vi "UHR-Fleezers Control (host) - 12.7e.vi"() -> ()   [LabVIEW 2012] (continued)
                      n1710 = Greater?(x=w2546, y="Stop F (pN) (mask)") -> (0:w2544:bool[])
                      n1711 = Or Array Elements(Boolean array=w2557) -> (logical OR=w2542:bool)
                      n1712 = Or Array Elements(Boolean array=w2544) -> (logical OR=w2541:bool)
                      n1713 = Greater?(x=w2551, y="Attempt Limit") -> (0:w2553:bool)
                      n1714 = case shown="True" w2553 {
                        frame False {
                        }
                        frame True {
                          n1715 = local write "Fish for Tether"(FALSE ("Fish for Tether")) -> ()
                          n1716 = call <vilib>:"Beep.vi"() -> ()  [unwired: 3 in, 9 out]
                          n1717 = local read "Messages"() -> (w2569:string)
                          n1718 = call "Update messages.vi"("Message to add"="Tether fishing timeout." ("Messages"), "Old message string"=w2569) -> ("New message string"=→"Messages":string)
                        }
                      }
                      n1719 = Select(t=w2542, s="Normal (on) or masked test (off)", f=w2541) -> (s? t:f=w2540:bool)
                    }
                  }
                  n1720 = local read "BD 2 Frequency 1 (MHz)"() -> (w2516:dbl)
                  n1721 = Select(t=w2517, s="Scan axis 2", f=w2516) -> (s? t:f=w2520:dbl)
                  n1722 = Add(x=w2508, y=w2520) -> (x+y=w2514:dbl)
                  n1723 = Select(t=w2514, s="Scan axis 2", f=w2517) -> (s? t:f=w2523:dbl)
                  n1724 = Select(t=w2516, s="Scan axis 2", f=w2514) -> (s? t:f=w2522:dbl)
                  n1725 = local read "BD 2 Frequency 2 (MHz)"() -> (w2525:dbl)
                  n1726 = local read "BD 2 Frequency 3 (MHz)"() -> (w2524:dbl)
                  n1727 = local read "Y RF Frequency Limits (MHz)"() -> (w2518:T16)
                  n1728 = local read "X RF Frequency Limits (MHz)"() -> (w2519:T16)
                  n1729 = local read "BD 1 Frequency 3 (MHz)"() -> (w2526:dbl)
                  n1730 = call "set RF board frequency - interlace.vi"("Board 2 Frequency Limits"=w2518, "Board 1 Frequency Limits"=w2519, "FPGA VI Reference In"=w2506, "Board 2 Frequency 3 (MHz)"=w2524, "Board 1 Frequency 3 (MHz)"=w2526, "Board 2 Frequency 2 (MHz)"=w2525, "Board 2 Frequency 1 (MHz)"=w2522, "Board 1 Frequency 2 (MHz)"=w2509, "Board 1 Frequency 1  (MHz)"=w2523) -> ()  [unwired: 1 in, 2 out]
                }
                frame #1 {
                  n1731 = And(x=w2577, y=w2574) -> (x .and. y?=w2576:bool)
                  n1732 = case "Only if were fishing and now formed tether" shown="True" w2576 {
                    tunnel: w2575 -> [w2579 w2594]
                    tunnel: [w2578 w2593] -> w2573
                    tunnel: w2572 -> [_ w2589]
                    frame False {
                      n1733 = local read "Fish for Tether"() -> (w2578:bool)
                      n1734 = case shown="False" w2578 {
                        tunnel: w2579 -> [w2580 _]
                        frame False {
                          n1735 = property on="BD 1 Frequency 1 (MHz)" class="DigNum (strict)"("Val(Sgnl)"=w2580) -> ()  [unwired: 2 in, 2 out]
                        }
                        frame True {
                        }
                      }
                    }
                    frame True {
                      w2593 = FALSE ("Fish for Tether")
                      n1736 = call <vilib>:"Beep.vi"() -> ()  [unwired: 3 in, 9 out]
                      n1737 = Number To Decimal String(number=w2589, width (-)=i16 1) -> (decimal integer string=w2587:string)
                      n1738 = Concatenate Strings("Formed tether in ", w2587, " attempt(s)." ("string")) -> (w2584:string)
                      n1739 = local read "Messages"() -> (w2591:string)
                      n1740 = local write "Fish for Tether"(w2593) -> ()
                      n1741 = call "Update messages.vi"("Message to add"=w2584, "Old message string"=w2591) -> ("New message string"=w2590:string)
                      n1742 = local write "Messages"(w2590) -> ()
                      n1743 = Get Date/Time In Seconds() -> (seconds since 1Jan1904=→"Time tether formed":timestamp)
                      n1744 = local read "Flow ON during cal?"() -> (w2581:bool)
                      n1745 = property on="Sample Channel\nFlow" class="Bool (strict)"("Val(Sgnl)"=w2581) -> (error out=w2582:errorcluster)  [unwired: 2 in, 1 out]
                      n1746 = case shown="\"2\", \"3\", \"4\", \"5\", \"6\"" "Then..." {
                        selector: "Then..." -> [_ w2597]
                        tunnel: w2594 -> [w2596 _]
                        tunnel: w2582 -> [_ _]
                        frame "1", Default {
                          n1747 = property on="BD 1 Frequency 1 (MHz)" class="DigNum (strict)"("Val(Sgnl)"=w2596) -> ()  [unwired: 2 in, 2 out]
                        }
                        frame "2", "3", "4", "5", "6" {
                          n1748 = flat-sequence {
                            tunnel: w2597 -> [w2599]
                            frame #0 {
                              n1749 = property on="Trap Delta (MHz)" class="DigNum (strict)"("Val(Sgnl)"="Move to Delta 1 (MHz)") -> ()  [unwired: 2 in, 2 out]
                            }
                            frame #1 {
                              n1750 = case shown="\"5\", \"6\"" w2599 {
                                selector: w2599 -> [w2602 w2612 _]
                                frame "3", "4" {
                                n1751 = flat-sequence {
                                tunnel: w2602 -> [w2603]
                                tunnel: [w2603] -> w2600
                                tunnel: [w2605] -> w2601
                                tunnel: w2600 -> [w2605]
                                tunnel: w2601 -> [w2609]
                                frame #0 {
                                n1752 = property on="Green Laser ON" class="Bool (strict)"("Val(Sgnl)"=TRUE ("Value (Signaling)")) -> ()  [unwired: 2 in, 2 out]
                                }
                                frame #1 {
                                n1753 = Multiply(x="Wait Before Save (s)", y=u32 1000 ("x")) -> (x*y=w2607:u32)
                                n1754 = Wait (ms)(milliseconds to wait=w2607) -> ()  [unwired: 1 out]
                                }
                                frame #2 {
                                n1755 = property on="Start Saving" class="Bool (strict)"("Value"=TRUE ("Start Saving")) -> ()  [unwired: 2 in, 2 out]
                                n1756 = case shown="\"4\"" w2609 {
                                frame Default {
                                }
                                frame "4" {
                                n1757 = property on="Fl. Triggered..." class="Bool (strict)"("Val(Sgnl)"=TRUE ("Value (Signaling)")) -> ()  [unwired: 2 in, 2 out]
                                }
                                }
                                }
                                }
                                }
                                frame "5", "6" {
                                n1758 = stacked-sequence {
                                tunnel: w2612 -> [_ _ _ _ _ _ w2624]
                                frame #0 {
                                n1759 = Replace Array Subset(array=u32[] [0] ("Index Values"), new element="Raster Set Upon Tether", index=0) -> (w2613:u32[])
                                n1760 = property on="Saved AOD Raster Scan Parameter Sets" class="Arr (strict)"("Index Values"=w2613) -> ()  [unwired: 2 in, 2 out]
                                }
                                frame #1 {
                                n1761 = Wait (ms)(milliseconds to wait=u32 500) -> ()  [unwired: 1 out]
                                }
                                frame #2 {
                                n1762 = property on="Load parameters" class="Bool (strict)"("Val(Sgnl)"=TRUE ("Value (Signaling)")) -> ()  [unwired: 2 in, 2 out]
                                n1763 = case shown="True" "Green ON During Raster" {
                                frame False {
                                }
                                frame True {
                                n1764 = property on="Green Laser ON" class="Bool (strict)"("Val(Sgnl)"=TRUE ("Value (Signaling)")) -> ()  [unwired: 2 in, 2 out]
                                }
                                }
                                }
                                frame #3 {
                                n1765 = Wait (ms)(milliseconds to wait=u32 500) -> ()  [unwired: 1 out]
                                }
                                frame #4 {
                                n1766 = property on="Trap Raster Scan" class="Bool (strict)"("Val(Sgnl)"=TRUE ("Value (Signaling)")) -> ()  [unwired: 2 in, 2 out]
                                }
                                frame #5 {
                                n1767 = Wait (ms)(milliseconds to wait=u32 2000) -> ()  [unwired: 1 out]
                                }
                                frame #6 {
                                n1768 = flat-sequence {
                                tunnel: w2624 -> [w2631]
                                frame #0 {
                                n1769 = while {
                                stop <- w2627 stop-if-true
                                n1770 = local read "Raster Scanning..."() -> (w2626:bool)
                                n1771 = local read "Saving..."() -> (w2629:bool)
                                n1772 = Wait (ms)(milliseconds to wait=u32 100) -> ()  [unwired: 1 out]
                                n1773 = Not(x=w2629) -> (.not. x?=w2628:bool)
                                n1774 = Not(x=w2626) -> (.not. x?=w2625:bool)
                                n1775 = And(x=w2628, y=w2625) -> (x .and. y?=w2627:bool)
                                }
                                }
                                frame #1 {
                                n1776 = local read "Tether"() -> (w2632:bool)
                                n1777 = case shown="True" w2632 {
                                tunnel: w2631 -> [_ w2634]
                                frame False {
                                n1778 = property on="Fish for Tether" class="Bool (strict)"("Val(Sgnl)"="Fish again after \nraster break?") -> ()  [unwired: 2 in, 2 out]
                                }
                                frame True {
                                n1779 = stacked-sequence {
                                tunnel: w2634 -> [_ w2638 _ _]
                                frame #0 {
                                n1780 = property on="Trap Delta (MHz)" class="DigNum (strict)"("Val(Sgnl)"="Move to Delta 2 (MHz)") -> ()  [unwired: 2 in, 2 out]
                                n1781 = case shown="True" "Flow ON after\ntether testing?" {
                                frame False {
                                }
                                frame True {
                                n1782 = property on="Sample Channel\nFlow" class="Bool (strict)"("Val(Sgnl)"=TRUE ("Value (Signaling)")) -> ()  [unwired: 2 in, 2 out]
                                }
                                }
                                }
                                frame #1 {
                                n1783 = flat-sequence {
                                tunnel: w2638 -> [w2640]
                                frame #0 {
                                n1784 = Wait (ms)(milliseconds to wait=u32 500) -> ()  [unwired: 1 out]
                                }
                                frame #1 {
                                n1785 = case shown="\"6\"" w2640 {
                                frame Default {
                                }
                                frame "6" {
                                n1786 = property on="Green Laser ON" class="Bool (strict)"("Val(Sgnl)"=TRUE ("Green Laser ON/Interlacing")) -> ()  [unwired: 2 in, 2 out]
                                }
                                }
                                }
                                frame #2 {
                                n1787 = Wait (ms)(milliseconds to wait=u32 500) -> ()  [unwired: 1 out]
                                }
                                frame #3 {
                                n1788 = local write "Start Saving"("Save at end (5, 6)") -> ()
                                }
                                }
                                }
                                frame #2 {
                                n1789 = local read "Bead Sep. Int. Time (s)"() -> (w2646:dbl)
                                n1790 = Multiply(x=w2646, y=1000.0) -> (x*y=w2645:dbl)
                                n1791 = Wait (ms)(milliseconds to wait=w2645) -> ()  [unwired: 1 out]
                                }
                                frame #3 {
                                n1792 = property on="Remove Offset" class="Bool (strict)"("Val(Sgnl)"=TRUE ("Value (Signaling)")) -> ()  [unwired: 2 in, 2 out]
                                }
                                }
                                }
                                }
                                }
                                }
                                }
                                }
                                }
                                frame "2", Default {
                                }
                              }
                            }
                          }
                        }
                      }
                      "Tether" <- "Tether Alarm?"
                    }
                  }
                }
                frame #2 {
                  n1793 = local read "Oscillate Set 1"() -> (w2653:bool)
                  n1794 = local read "Stop All"() -> (w2651:bool)
                  n1795 = Or(x=w2653, y=w2648) -> (x .or. y?=w2650:bool)
                  n1796 = Not(x=w2650) -> (.not. x?=w2652:bool)
                  n1797 = Compound Arithmetic op=OR(w2651, w2652) -> (w2649:bool)
                }
              }
              n1798 = node-c288() -> ()  [unwired: 2 out]
            }
            n1799 = node-c288(w2485) -> ()  [unwired: 1 out]
          }
        }
      }
      event "Fl. Triggered...": Value Change {
        n1800 = event-data() -> ()  [unwired: 7 out]
        n1801 = case shown="True" "Fl. Triggered..." {
          frame False {
          }
          frame True {
            n1802 = node-c288() -> (w2664:T23)  [unwired: 4 out]
            n1803 = timed-loop {
              timing: w2664 -> [_]
              timing-out: [_] -> w2663
              tunnel: "Action" -> [w2672]
              shift-right: [w2669] -> _
              shift-left: u8 255 -> [w2671]
              shift-right: [w2666] -> _
              shift-left: 255 -> [w2668]
              stop <- w2665 stop-if-true
              # "Reset confocal spot"
              n1804 = node-c288() -> ()  [unwired: 2 out]
              n1805 = flat-sequence {
                tunnel: w2672 -> [w2692]
                tunnel: w2671 -> [w2691]
                tunnel: [w2690] -> w2670
                tunnel: w2668 -> [w2677]
                tunnel: [w2676] -> w2667
                tunnel: [w3071] -> w2665
                tunnel: w2670 -> [w3070]
                tunnel: [w3070] -> w2669
                tunnel: [w3069] -> w2666
                tunnel: w2667 -> [w3069]
                frame #0 {
                  n1806 = local read "Delta Fl. 2"() -> (w2689:dbl)
                  n1807 = local read "Delta Fl. 1"() -> (w2684:dbl)
                  n1808 = Multiply(x="Fl. Delta Thresh. (kHz)", y=1000.0) -> (x*y=w2679:dbl)
                  n1809 = Select(t=w2684, s="APD to Watch", f=w2689) -> (s? t:f=w2680:dbl)
                  n1810 = Greater?(x=w2680, y=w2679) -> (0:w2685:bool)
                  n1811 = Or(x="Force Yank", y=w2685) -> (x .or. y?=w2683:bool)
                  n1812 = And(x=w2683, y="Yank when?") -> (x .and. y?=w2681:bool)
                  n1813 = case shown="False" w2681 {
                    tunnel: w2692 -> [w2695 w2896]
                    tunnel: w2691 -> [w2697 w2892]
                    tunnel: [w2697 w2890] -> w2690
                    tunnel: w2680 -> [w2703 _]
                    tunnel: w2679 -> [w2702 _]
                    tunnel: "Force Yank" -> [w2700 _]
                    tunnel: w2677 -> [w2699 w2889]
                    tunnel: [w2698 w2889] -> w2676
                    frame False {
                      n1814 = Negate(x=w2702) -> (-x=w2694:dbl)
                      n1815 = local write "Fl. High"(TRUE ("Fl. High")) -> ()
                      n1816 = Less?(x=w2703, y=w2694) -> (x < y?=w2701:bool)
                      n1817 = Or(x=w2700, y=w2701) -> (x .or. y?=w2696:bool)
                      n1818 = case shown="True" w2696 {
                        tunnel: w2699 -> [w2704 w2714]
                        tunnel: [w2704 w2713] -> w2698
                        tunnel: w2695 -> [_ w2712]
                        frame False {
                        }
                        frame True {
                          n1819 = flat-sequence {
                            tunnel: w2714 -> [w2720]
                            tunnel: w2712 -> [w2717]
                            tunnel: [w2719] -> w2711
                            tunnel: [w2718] -> w2710
                            tunnel: [w2717] -> w2709
                            tunnel: w2708 -> [w2716]
                            tunnel: [w2716] -> w2707
                            tunnel: w2706 -> [w2715]
                            tunnel: [w2715] -> w2705
                            tunnel: [w2791] -> w2713
                            tunnel: w2711 -> [w2791]
                            tunnel: w2710 -> [w2790]
                            tunnel: w2709 -> [w2789]
                            tunnel: w2707 -> [w2788]
                            tunnel: w2705 -> [w2787]
                            frame #0 {
                              n1820 = call <vilib>:"Beep.vi"() -> ()  [unwired: 12 in]
                              n1821 = local write "Waiting"(FALSE ("Waiting")) -> ()
                              n1822 = Increment(x=w2720) -> (x+1=w2719:i32)
                              n1823 = case shown="\"Image\"" w2717 {
                                tunnel: w2719 -> [_ w2725 _]
                                frame "Alarm", Default {
                                }
                                frame "Yank" {
                                n1824 = flat-sequence {
                                tunnel: w2725 -> [w2728]
                                tunnel: [w2727] -> w2724
                                tunnel: [w2726] -> w2723
                                tunnel: w2724 -> [w2738]
                                tunnel: w2723 -> [w2739]
                                frame #0 {
                                n1825 = local read "Yank Delay (s)"() -> (w2731:dbl)
                                n1826 = local read "N Array El"() -> (w2726:u8)
                                n1827 = Quotient & Remainder(x=w2728, y=w2726) -> (x-y*floor(x/y)=w2727:i32)  [unwired: 1 out]
                                n1828 = Multiply(x=w2731, y=1000.0) -> (x*y=w2729:dbl)
                                n1829 = Wait (ms)(milliseconds to wait=w2729) -> ()  [unwired: 1 out]
                                }
                                frame #1 {
                                n1830 = local read "Yank to which?"() -> (w2733:bool)
                                n1831 = local read "Random Choice"() -> (w2743:bool)
                                n1832 = local read "Yank to Trap Delta (MHz)"() -> (w2736:dbl[])
                                n1833 = local read "Yank to SP"() -> (w2737:dbl[])
                                n1834 = Random Number (0-1)() -> (number: 0 to 1=w2742:dbl)
                                n1835 = Multiply(x=w2739, y=w2742) -> (x*y=w2741:dbl)
                                n1836 = Round Toward -Infinity(1:w2741) -> (0:w2740:dbl)
                                n1837 = Select(t=w2740, s=w2743, f=w2738) -> (s? t:f=w2734:dbl)
                                n1838 = Select(t=w2736, s=w2733, f=w2737) -> (s? t:f=w2735:dbl[])
                                n1839 = Index Array(array=w2735, index=w2734) -> (element=w2732:dbl)
                                n1840 = case shown="True" w2733 {
                                tunnel: w2732 -> [w2744 w2771]
                                frame False {
                                n1841 = flat-sequence {
                                tunnel: w2744 -> [w2745]
                                frame #0 {
                                n1842 = property on="Trap Pos FB SP" class="DigNum (strict)"("Val(Sgnl)"=w2745) -> ()  [unwired: 2 in, 2 out]
                                }
                                frame #1 {
                                n1843 = Wait (ms)(milliseconds to wait=u32 700) -> ()  [unwired: 1 out]
                                }
                                frame #2 {
                                n1844 = local read "Action (%)"() -> (w2750:dbl)
                                n1845 = Absolute Value(x=w2750) -> (abs(x)=w2749:dbl)
                                n1846 = Greater?(x=w2749, y=70.0) -> (0:w2747:bool)
                                n1847 = property on="Remove Action Offset" class="Bool (strict)"("Val(Sgnl)"=w2747) -> ()  [unwired: 2 in, 2 out]
                                }
                                frame #3 {
                                n1848 = for {
                                N: 4 -> [_]
                                n1849 = flat-sequence {
                                frame #0 {
                                n1850 = Wait (ms)(milliseconds to wait=u32 500) -> ()  [unwired: 1 out]
                                }
                                frame #1 {
                                n1851 = local read "Action (%)"() -> (w2756:dbl)
                                n1852 = Absolute Value(x=w2756) -> (abs(x)=w2755:dbl)
                                n1853 = Greater?(x=w2755, y=70.0) -> (0:w2753:bool)
                                n1854 = property on="Remove Action Offset" class="Bool (strict)"("Val(Sgnl)"=w2753) -> ()  [unwired: 2 in, 2 out]
                                }
                                }
                                }
                                }
                                frame #4 {
                                n1855 = Wait (ms)(milliseconds to wait=u32 500) -> ()  [unwired: 1 out]
                                }
                                frame #5 {
                                n1856 = local read "Mean"() -> (w2764:dbl)
                                n1857 = Greater?(x=w2764, y=11.0) -> (0:w2758:bool)
                                n1858 = Not(x=w2758) -> (.not. x?=w2759:bool)
                                n1859 = And(x=w2759, y="Shift confocal") -> (x .and. y?=w2761:bool)
                                n1860 = And(x=w2758, y="Shift confocal") -> (x .and. y?=w2762:bool)
                                n1861 = case shown="True" w2762 {
                                frame False {
                                }
                                frame True {
                                n1862 = local read "Confocal Y 2 (V)"() -> (w2768:dbl)
                                n1863 = local read "Confocal X 2 (V)"() -> (w2767:dbl)
                                n1864 = property on="AO1" class="Slide (strict)"("Val(Sgnl)"=w2768) -> ()  [unwired: 2 in, 2 out]
                                n1865 = property on="AO2" class="Slide (strict)"("Val(Sgnl)"=w2767) -> ()  [unwired: 2 in, 2 out]
                                }
                                }
                                n1866 = case shown="True" w2761 {
                                frame False {
                                }
                                frame True {
                                n1867 = local read "Confocal Y 1 (V)"() -> (w2766:dbl)
                                n1868 = local read "Confocal X 1 (V)"() -> (w2765:dbl)
                                n1869 = property on="AO1" class="Slide (strict)"("Val(Sgnl)"=w2766) -> ()  [unwired: 2 in, 2 out]
                                n1870 = property on="AO2" class="Slide (strict)"("Val(Sgnl)"=w2765) -> ()  [unwired: 2 in, 2 out]
                                }
                                }
                                }
                                frame #6 {
                                n1871 = Wait (ms)(milliseconds to wait=u32 1500) -> ()  [unwired: 1 out]
                                }
                                frame #7 {
                                n1872 = property on="Rem fb disp offset" class="Bool (strict)"("Val(Sgnl)"=TRUE ("Value (Signaling)")) -> ()  [unwired: 2 in, 2 out]
                                }
                                }
                                }
                                frame True {
                                n1873 = flat-sequence {
                                tunnel: w2771 -> [w2772]
                                frame #0 {
                                n1874 = property on="Trap Delta (MHz)" class="DigNum (strict)"("Val(Sgnl)"=w2772) -> ()  [unwired: 2 in, 2 out]
                                }
                                frame #1 {
                                n1875 = Wait (ms)(milliseconds to wait=u32 500) -> ()  [unwired: 1 out]
                                }
                                frame #2 {
                                n1876 = local read "Shift confocal"() -> (w2778:bool)
                                n1877 = local read "Mean"() -> (w2780:dbl)
                                n1878 = Greater?(x=w2780, y=11.0) -> (0:w2777:bool)
                                n1879 = Not(x=w2777) -> (.not. x?=w2776:bool)
                                n1880 = And(x=w2776, y=w2778) -> (x .and. y?=w2774:bool)
                                n1881 = And(x=w2777, y=w2778) -> (x .and. y?=w2775:bool)
                                n1882 = case shown="True" w2775 {
                                frame False {
                                }
                                frame True {
                                n1883 = local read "Confocal Y 2 (V)"() -> (w2784:dbl)
                                n1884 = local read "Confocal X 2 (V)"() -> (w2783:dbl)
                                n1885 = property on="AO2" class="Slide (strict)"("Val(Sgnl)"=w2783) -> ()  [unwired: 2 in, 2 out]
                                n1886 = property on="AO1" class="Slide (strict)"("Val(Sgnl)"=w2784) -> ()  [unwired: 2 in, 2 out]
                                }
                                }
                                n1887 = case shown="True" w2774 {
                                frame False {
                                }
                                frame True {
                                n1888 = local read "Confocal X 1 (V)"() -> (w2781:dbl)
                                n1889 = local read "Confocal Y 1 (V)"() -> (w2782:dbl)
                                n1890 = property on="AO2" class="Slide (strict)"("Val(Sgnl)"=w2781) -> ()  [unwired: 2 in, 2 out]
                                n1891 = property on="AO1" class="Slide (strict)"("Val(Sgnl)"=w2782) -> ()  [unwired: 2 in, 2 out]
                                }
                                }
                                }
                                }
                                }
                                }
                                }
                                }
                                }
                                frame "Image" {
                                n1892 = property on="Confocal Image" class="Bool (strict)"("Val(Sgnl)"=TRUE ("Value (Signaling)")) -> ()  [unwired: 2 in, 2 out]
                                }
                              }
                              n1893 = local write "Fl. High"(FALSE ("Fl. High")) -> ()
                              n1894 = local read "Time (s)"() -> (w2718:dbl)
                            }
                            frame #1 {
                              n1895 = case shown="True" "Auto F Reset" {
                                tunnel: w2790 -> [_ w2795]
                                tunnel: w2789 -> [_ w2794]
                                tunnel: w2788 -> [_ w2793]
                                tunnel: w2787 -> [_ w2792]
                                frame False {
                                }
                                frame True {
                                n1896 = node-c288() -> (w2797:T23)  [unwired: 4 in]
                                n1897 = timed-loop {
                                timing: w2797 -> [_]
                                timing-out: [_] -> w2796
                                tunnel: w2795 -> [w2802]
                                tunnel: w2794 -> [w2801]
                                tunnel: w2793 -> [w2800]
                                tunnel: w2792 -> [w2799]
                                stop <- w2798 stop-if-true
                                n1898 = node-c288() -> ()  [unwired: 1 in, 1 out]
                                n1899 = local read "Fl. Delta Thresh. (kHz)"() -> (w2811:dbl)
                                n1900 = local read "APD to Watch"() -> (w2812:bool)
                                n1901 = local read "Delta Fl. 1"() -> (w2813:dbl)
                                n1902 = local read "Delta Fl. 2"() -> (w2814:dbl)
                                n1903 = local read "Fl. Triggered..."() -> (w2805:bool)
                                n1904 = local read "Stop All"() -> (w2806:bool)
                                n1905 = local read "Reset Force"() -> (w2804:bool)
                                n1906 = Multiply(x=w2811, y=1000.0) -> (x*y=w2809:dbl)
                                n1907 = Select(t=w2813, s=w2812, f=w2814) -> (s? t:f=w2808:dbl)
                                n1908 = Not(x=w2805) -> (.not. x?=w2803:bool)
                                n1909 = Greater?(x=w2808, y=w2809) -> (0:w2807:bool)
                                n1910 = Compound Arithmetic op=OR(w2807, w2806, w2803, w2804) -> (w2798:bool)
                                n1911 = case shown="True" w2798 {
                                tunnel: w2802 -> [_ w2818]
                                tunnel: w2801 -> [_ w2822]
                                tunnel: w2800 -> [_ w2821]
                                tunnel: w2799 -> [_ w2820]
                                frame False {
                                }
                                frame True {
                                n1912 = case shown="\"Yank\"" w2822 {
                                tunnel: w2821 -> [_ w2832]
                                tunnel: w2820 -> [_ w2830]
                                frame "Image", Default {
                                }
                                frame "Yank" {
                                n1913 = flat-sequence {
                                tunnel: [w2835] -> w2833
                                tunnel: w2832 -> [w2835]
                                tunnel: [w2834] -> w2831
                                tunnel: w2830 -> [w2834]
                                tunnel: w2833 -> [w2841]
                                tunnel: w2831 -> [w2839]
                                frame #0 {
                                n1914 = local read "Yank Delay (s)"() -> (w2838:dbl)
                                n1915 = Multiply(x=w2838, y=1000.0) -> (x*y=w2836:dbl)
                                n1916 = Wait (ms)(milliseconds to wait=w2836) -> ()  [unwired: 1 out]
                                }
                                frame #1 {
                                n1917 = local read "Yank to which?"() -> (w2840:bool)
                                n1918 = case shown="False" w2840 {
                                tunnel: w2841 -> [_ w2869]
                                tunnel: w2839 -> [w2842 _]
                                frame False {
                                n1919 = flat-sequence {
                                tunnel: w2842 -> [w2843]
                                frame #0 {
                                n1920 = property on="Trap Pos FB SP" class="DigNum (strict)"("Val(Sgnl)"=w2843) -> ()  [unwired: 2 in, 2 out]
                                }
                                frame #1 {
                                n1921 = Wait (ms)(milliseconds to wait=u32 700) -> ()  [unwired: 1 out]
                                }
                                frame #2 {
                                n1922 = local read "Action (%)"() -> (w2848:dbl)
                                n1923 = Absolute Value(x=w2848) -> (abs(x)=w2847:dbl)
                                n1924 = Greater?(x=w2847, y=70.0) -> (0:w2845:bool)
                                n1925 = property on="Remove Action Offset" class="Bool (strict)"("Val(Sgnl)"=w2845) -> ()  [unwired: 2 in, 2 out]
                                }
                                frame #3 {
                                n1926 = for {
                                N: 4 -> [_]
                                n1927 = flat-sequence {
                                frame #0 {
                                n1928 = Wait (ms)(milliseconds to wait=u32 500) -> ()  [unwired: 1 out]
                                }
                                frame #1 {
                                n1929 = local read "Action (%)"() -> (w2854:dbl)
                                n1930 = Absolute Value(x=w2854) -> (abs(x)=w2853:dbl)
                                n1931 = Greater?(x=w2853, y=70.0) -> (0:w2851:bool)
                                n1932 = property on="Remove Action Offset" class="Bool (strict)"("Val(Sgnl)"=w2851) -> ()  [unwired: 2 in, 2 out]
                                }
                                }
                                }
                                }
                                frame #4 {
                                n1933 = Wait (ms)(milliseconds to wait=u32 500) -> ()  [unwired: 1 out]
                                }
                                frame #5 {
                                n1934 = local read "Shift confocal"() -> (w2859:bool)
                                n1935 = local read "Mean"() -> (w2862:dbl)
                                n1936 = Greater?(x=w2862, y=11.0) -> (0:w2858:bool)
                                n1937 = Not(x=w2858) -> (.not. x?=w2857:bool)
                                n1938 = And(x=w2858, y=w2859) -> (x .and. y?=w2860:bool)
                                n1939 = And(x=w2857, y=w2859) -> (x .and. y?=w2856:bool)
                                n1940 = case shown="True" w2860 {
                                frame False {
                                }
                                frame True {
                                n1941 = local read "Confocal X 2 (V)"() -> (w2865:dbl)
                                n1942 = local read "Confocal Y 2 (V)"() -> (w2866:dbl)
                                n1943 = property on="AO2" class="Slide (strict)"("Val(Sgnl)"=w2865) -> ()  [unwired: 2 in, 2 out]
                                n1944 = property on="AO1" class="Slide (strict)"("Val(Sgnl)"=w2866) -> ()  [unwired: 2 in, 2 out]
                                }
                                }
                                n1945 = case shown="True" w2856 {
                                frame False {
                                }
                                frame True {
                                n1946 = local read "Confocal Y 1 (V)"() -> (w2864:dbl)
                                n1947 = local read "Confocal X 1 (V)"() -> (w2863:dbl)
                                n1948 = property on="AO1" class="Slide (strict)"("Val(Sgnl)"=w2864) -> ()  [unwired: 2 in, 2 out]
                                n1949 = property on="AO2" class="Slide (strict)"("Val(Sgnl)"=w2863) -> ()  [unwired: 2 in, 2 out]
                                }
                                }
                                }
                                frame #6 {
                                n1950 = Wait (ms)(milliseconds to wait=u32 1500) -> ()  [unwired: 1 out]
                                }
                                frame #7 {
                                n1951 = property on="Rem fb disp offset" class="Bool (strict)"("Val(Sgnl)"=TRUE ("Value (Signaling)")) -> ()  [unwired: 2 in, 2 out]
                                }
                                }
                                }
                                frame True {
                                n1952 = flat-sequence {
                                tunnel: w2869 -> [w2870]
                                frame #0 {
                                n1953 = property on="Trap Delta (MHz)" class="DigNum (strict)"("Val(Sgnl)"=w2870) -> ()  [unwired: 2 in, 2 out]
                                }
                                frame #1 {
                                n1954 = Wait (ms)(milliseconds to wait=u32 500) -> ()  [unwired: 1 out]
                                }
                                frame #2 {
                                n1955 = local read "Shift confocal"() -> (w2876:bool)
                                n1956 = local read "Mean"() -> (w2877:dbl)
                                n1957 = Greater?(x=w2877, y=11.0) -> (0:w2875:bool)
                                n1958 = And(x=w2875, y=w2876) -> (x .and. y?=w2873:bool)
                                n1959 = Not(x=w2875) -> (.not. x?=w2874:bool)
                                n1960 = And(x=w2874, y=w2876) -> (x .and. y?=w2872:bool)
                                n1961 = case shown="True" w2873 {
                                frame False {
                                }
                                frame True {
                                n1962 = local read "Confocal Y 2 (V)"() -> (w2882:dbl)
                                n1963 = local read "Confocal X 2 (V)"() -> (w2881:dbl)
                                n1964 = property on="AO1" class="Slide (strict)"("Val(Sgnl)"=w2882) -> ()  [unwired: 2 in, 2 out]
                                n1965 = property on="AO2" class="Slide (strict)"("Val(Sgnl)"=w2881) -> ()  [unwired: 2 in, 2 out]
                                }
                                }
                                n1966 = case shown="True" w2872 {
                                frame False {
                                }
                                frame True {
                                n1967 = local read "Confocal Y 1 (V)"() -> (w2880:dbl)
                                n1968 = local read "Confocal X 1 (V)"() -> (w2879:dbl)
                                n1969 = property on="AO2" class="Slide (strict)"("Val(Sgnl)"=w2879) -> ()  [unwired: 2 in, 2 out]
                                n1970 = property on="AO1" class="Slide (strict)"("Val(Sgnl)"=w2880) -> ()  [unwired: 2 in, 2 out]
                                }
                                }
                                }
                                }
                                }
                                }
                                }
                                }
                                }
                                }
                                n1971 = local read "Time (s)"() -> (w2817:dbl)
                                n1972 = Subtract(x=w2818, y=w2817) -> (x-y=w2829:dbl)
                                n1973 = Number To Decimal String(number=w2829, width (-)=i16 0) -> (decimal integer string=w2827:string)
                                n1974 = Concatenate Strings(w2827, " s fluorescence event") -> (w2824:string)
                                n1975 = local read "Messages"() -> (w2825:string)
                                n1976 = local write "Duration (s)"(w2829) -> ()
                                n1977 = call "Update messages.vi"("Message to add"=w2824, "Old message string"=w2825) -> ("New message string"=w2823:string)
                                n1978 = local write "Messages"(w2823) -> ()
                                n1979 = call <vilib>:"Beep.vi"() -> ()  [unwired: 12 in]
                                n1980 = local write "Reset Force"(FALSE ("Force Reset")) -> ()
                                n1981 = local write "Fl. High"(TRUE ("Fl. High")) -> ()
                                n1982 = local write "Waiting"(TRUE ("Waiting")) -> ()
                                }
                                }
                                n1983 = node-c288() -> ()  [unwired: 1 in, 1 out]
                                }
                                n1984 = node-c288(w2796) -> ()  [unwired: 1 out]
                                }
                              }
                            }
                          }
                          n1985 = local read "Trap Delta (MHz)"() -> (w2708:dbl)
                          n1986 = local read "Trap Pos FB SP"() -> (w2706:fxp<+/-,16,1>)
                        }
                      }
                    }
                    frame True {
                      n1987 = flat-sequence {
                        tunnel: w2893 -> [w2903]
                        tunnel: [w2903] -> w2897
                        tunnel: w2896 -> [w2902]
                        tunnel: [w2902] -> w2895
                        tunnel: [w2901] -> w2894
                        tunnel: w2892 -> [w2900]
                        tunnel: [w2899] -> w2891
                        tunnel: w2888 -> [w2898]
                        tunnel: [w2898] -> w2887
                        tunnel: w2897 -> [w2973]
                        tunnel: w2895 -> [w2972]
                        tunnel: w2894 -> [w2971]
                        tunnel: w2891 -> [w2970]
                        tunnel: w2887 -> [w2969]
                        tunnel: [w2970] -> w2890
                        frame #0 {
                          n1988 = call <vilib>:"Beep.vi"() -> ()  [unwired: 3 in, 9 out]
                          n1989 = local write "Waiting"(FALSE ("Waiting")) -> ()
                          n1990 = Increment(x=w2900) -> (x+1=w2899:u8)
                          n1991 = case shown="\"Yank\"" w2902 {
                            tunnel: w2899 -> [_ _ w2909]
                            frame "Image" {
                              n1992 = property on="Confocal Image" class="Bool (strict)"("Val(Sgnl)"=TRUE ("Value (Signaling)")) -> ()  [unwired: 2 in, 2 out]
                            }
                            frame "Alarm", Default {
                            }
                            frame "Yank" {
                              n1993 = flat-sequence {
                                tunnel: w2909 -> [w2912]
                                tunnel: [w2911] -> w2908
                                tunnel: ["N Array El"] -> w2907
                                tunnel: w2908 -> [w2926]
                                tunnel: w2907 -> [w2922]
                                frame #0 {
                                n1994 = Multiply(x="Yank Delay (s)", y=1000.0) -> (x*y=w2915:dbl)
                                n1995 = Quotient & Remainder(x=w2912, y="N Array El") -> (x-y*floor(x/y)=w2911:u8)  [unwired: 1 out]
                                n1996 = Wait (ms)(milliseconds to wait=w2915) -> ()  [unwired: 1 out]
                                }
                                frame #1 {
                                n1997 = Random Number (0-1)() -> (number: 0 to 1=w2923:dbl)
                                n1998 = Multiply(x=w2922, y=w2923) -> (x*y=w2921:dbl)
                                n1999 = Round Toward -Infinity(1:w2921) -> (0:w2920:dbl)
                                n2000 = Select(t=w2920, s="Random Choice", f=w2926) -> (s? t:f=w2924:dbl)
                                n2001 = Select(t="Yank to Trap Delta (MHz)", s="Yank to which?", f="Yank to SP") -> (s? t:f=w2917:dbl[])
                                n2002 = Index Array(array=w2917, index=w2924) -> (element=w2927:dbl)
                                n2003 = case shown="False" "Yank to which?" {
                                tunnel: w2927 -> [w2928 w2954]
                                frame False {
                                n2004 = flat-sequence {
                                tunnel: w2928 -> [w2929]
                                frame #0 {
                                n2005 = property on="Trap Pos FB SP" class="DigNum (strict)"("Val(Sgnl)"=w2929) -> ()  [unwired: 2 in, 2 out]
                                }
                                frame #1 {
                                n2006 = Wait (ms)(milliseconds to wait=u32 700) -> ()  [unwired: 1 out]
                                }
                                frame #2 {
                                n2007 = local read "Action (%)"() -> (w2934:dbl)
                                n2008 = Absolute Value(x=w2934) -> (abs(x)=w2933:dbl)
                                n2009 = Greater?(x=w2933, y=70.0) -> (0:w2931:bool)
                                n2010 = property on="Remove Action Offset" class="Bool (strict)"("Val(Sgnl)"=w2931) -> ()  [unwired: 2 in, 2 out]
                                }
                                frame #3 {
                                n2011 = for {
                                N: 4 -> [_]
                                n2012 = flat-sequence {
                                frame #0 {
                                n2013 = Wait (ms)(milliseconds to wait=u32 500) -> ()  [unwired: 1 out]
                                }
                                frame #1 {
                                n2014 = local read "Action (%)"() -> (w2940:dbl)
                                n2015 = Absolute Value(x=w2940) -> (abs(x)=w2939:dbl)
                                n2016 = Greater?(x=w2939, y=70.0) -> (0:w2937:bool)
                                n2017 = property on="Remove Action Offset" class="Bool (strict)"("Val(Sgnl)"=w2937) -> ()  [unwired: 2 in, 2 out]
                                }
                                }
                                }
                                }
                                frame #4 {
                                n2018 = local read "Shift confocal"() -> (w2944:bool)
                                n2019 = local read "Mean"() -> (w2947:dbl)
                                n2020 = Greater?(x=w2947, y=11.0) -> (0:w2943:bool)
                                n2021 = Not(x=w2943) -> (.not. x?=w2942:bool)
                                n2022 = And(x=w2942, y=w2944) -> (x .and. y?=w2941:bool)
                                n2023 = And(x=w2943, y=w2944) -> (x .and. y?=w2945:bool)
                                n2024 = case shown="True" w2945 {
                                frame False {
                                }
                                frame True {
                                n2025 = local read "Confocal X 2 (V)"() -> (w2950:dbl)
                                n2026 = local read "Confocal Y 2 (V)"() -> (w2951:dbl)
                                n2027 = property on="AO2" class="Slide (strict)"("Val(Sgnl)"=w2950) -> ()  [unwired: 2 in, 2 out]
                                n2028 = property on="AO1" class="Slide (strict)"("Val(Sgnl)"=w2951) -> ()  [unwired: 2 in, 2 out]
                                }
                                }
                                n2029 = case shown="True" w2941 {
                                frame False {
                                }
                                frame True {
                                n2030 = local read "Confocal X 1 (V)"() -> (w2948:dbl)
                                n2031 = local read "Confocal Y 1 (V)"() -> (w2949:dbl)
                                n2032 = property on="AO1" class="Slide (strict)"("Val(Sgnl)"=w2949) -> ()  [unwired: 2 in, 2 out]
                                n2033 = property on="AO2" class="Slide (strict)"("Val(Sgnl)"=w2948) -> ()  [unwired: 2 in, 2 out]
                                }
                                }
                                }
                                frame #5 {
                                n2034 = Wait (ms)(milliseconds to wait=u32 1500) -> ()  [unwired: 1 out]
                                }
                                frame #6 {
                                n2035 = property on="Rem fb disp offset" class="Bool (strict)"("Val(Sgnl)"=TRUE ("Value (Signaling)")) -> ()  [unwired: 2 in, 2 out]
                                }
                                }
                                }
                                frame True {
                                n2036 = flat-sequence {
                                tunnel: w2954 -> [w2955]
                                frame #0 {
                                n2037 = property on="Trap Delta (MHz)" class="DigNum (strict)"("Val(Sgnl)"=w2955) -> ()  [unwired: 2 in, 2 out]
                                }
                                frame #1 {
                                n2038 = Wait (ms)(milliseconds to wait=u32 500) -> ()  [unwired: 1 out]
                                }
                                frame #2 {
                                n2039 = local read "Shift confocal"() -> (w2959:bool)
                                n2040 = local read "Mean"() -> (w2957:dbl)
                                n2041 = Greater?(x=w2957, y=11.0) -> (0:w2960:bool)
                                n2042 = Not(x=w2960) -> (.not. x?=w2961:bool)
                                n2043 = And(x=w2961, y=w2959) -> (x .and. y?=w2963:bool)
                                n2044 = And(x=w2960, y=w2959) -> (x .and. y?=w2962:bool)
                                n2045 = case shown="True" w2962 {
                                frame False {
                                }
                                frame True {
                                n2046 = local read "Confocal Y 2 (V)"() -> (w2967:dbl)
                                n2047 = local read "Confocal X 2 (V)"() -> (w2966:dbl)
                                n2048 = property on="AO1" class="Slide (strict)"("Val(Sgnl)"=w2967) -> ()  [unwired: 2 in, 2 out]
                                n2049 = property on="AO2" class="Slide (strict)"("Val(Sgnl)"=w2966) -> ()  [unwired: 2 in, 2 out]
                                }
                                }
                                n2050 = case shown="True" w2963 {
                                frame False {
                                }
                                frame True {
                                n2051 = local read "Confocal X 1 (V)"() -> (w2964:dbl)
                                n2052 = local read "Confocal Y 1 (V)"() -> (w2965:dbl)
                                n2053 = property on="AO2" class="Slide (strict)"("Val(Sgnl)"=w2964) -> ()  [unwired: 2 in, 2 out]
                                n2054 = property on="AO1" class="Slide (strict)"("Val(Sgnl)"=w2965) -> ()  [unwired: 2 in, 2 out]
                                }
                                }
                                }
                                }
                                }
                                }
                                }
                              }
                            }
                          }
                          n2055 = local read "Time (s)"() -> (w2901:dbl)
                          "Fl. High" <- TRUE ("Yanking")
                        }
                        frame #1 {
                          n2056 = local read "Auto F Reset"() -> (w2968:bool)
                          n2057 = case shown="True" w2968 {
                            tunnel: w2973 -> [_ w2977]
                            tunnel: w2972 -> [_ w2976]
                            tunnel: w2971 -> [_ w2975]
                            tunnel: w2969 -> [_ w2974]
                            frame False {
                            }
                            frame True {
                              n2058 = node-c288() -> (w2979:T23)  [unwired: 4 out]
                              n2059 = timed-loop {
                                timing: w2979 -> [_]
                                timing-out: [_] -> w2978
                                tunnel: w2977 -> [w2997]
                                tunnel: w2976 -> [w2996]
                                tunnel: w2975 -> [w2995]
                                tunnel: w2974 -> [w2994]
                                stop <- w2980 stop-if-true
                                n2060 = node-c288() -> ()  [unwired: 2 out]
                                n2061 = local read "Fl. Delta Thresh. (kHz)"() -> (w2988:dbl)
                                n2062 = local read "Fl. Triggered..."() -> (w2993:bool)